vi "HFRR ADV v040 new software.vi"() -> ()   [LabVIEW 2025] (continued)
                    n2637 = Number To Fractional String(number=w3230, width (-)=i16 9 ("precision (6)"), precision (6)=i16 3) -> (F-format string=w3231:string)  [unwired: 1 in]
                    n2638 = Number To Fractional String(number=w3227, width (-)=i16 9 ("precision (6)"), precision (6)=i16 3) -> (F-format string=w3226:string)  [unwired: 1 in]
                    n2639 = Number To Fractional String(number=w3218, width (-)=i16 9 ("precision (6)"), precision (6)=i16 6) -> (F-format string=w3253:string)  [unwired: 1 in]
                    n2640 = Number To Fractional String(number=w3252, width (-)=i16 14 ("precision (6)"), precision (6)=i16 3) -> (F-format string=w3254:string)  [unwired: 1 in]
                    n2641 = Bundle("y"=1.02, "LVDT STROKE DISPLAY"=w3199, "y"=0.98) -> (w3219:T31)  [unwired: 1 in]
                    n2642 = Number To Fractional String(number="Ambient Humidity :", width (-)=i16 9 ("precision (6)"), precision (6)=i16 6) -> (F-format string=w3211:string)  [unwired: 1 in]
                    n2643 = local read "RUN"() -> (w3217:bool)
                    n2644 = case shown="True" w3217 {
                      tunnel: w3219 -> [_ w3270]
                      tunnel: w3199 -> [_ w3269]
                      tunnel: w3199 -> [_ w3267]
                      tunnel: w3199 -> [_ w3268]
                      frame False {
                      }
                      frame True {
                        "Stroke ( mm )" <- w3270
                        "Stroke ( mm )" <- w3270
                        "Stroke 4" <- w3269
                        "Stroke 3" <- w3267
                        "Stroke 2" <- w3268
                        "measured_stroke" <- w3267
                      }
                    }
                    n2645 = Concatenate Strings(w3254, w3213, w3253, w3213, w3245, w3213, w3244, w3213, w3241, w3213, w3238, w3213, w3235, w3213, w3231, w3213, w3226, w3213, w3211, "\r") -> (w3251:string)
                    n2646 = call <vilib>:"Write Characters To File.vi"("append to file? (new file:F)"=TRUE, "character string"=w3251, "file path (dialog if empty)"=w3204) -> ()  [unwired: 2 in, 1 out]
                    "refresh flag" <- TRUE ("refresh flag")
                    "LVDT STROKE Actual" <- w3197
                  }
                }
                n2647 = case shown="True" w3113 {
                  tunnel: w3123 -> [_ w3149]
                  tunnel: w3128 -> [_ w3159]
                  tunnel: [0.0 w3155] -> _
                  tunnel: w3122 -> [_ w3154]
                  tunnel: [0.0 w3153] -> _
                  tunnel: w3112 -> [_ w3153]
                  tunnel: w3126 -> [w3142 _]
                  frame False {
                    n2648 = local write "acq timer"(w3142) -> ()
                    n2649 = local write "Test Duration Status"(0.0 ("Test Duration Status")) -> ()
                  }
                  frame True {
                    n2650 = local read "Set Hz"() -> (w3156:dbl)
                    n2651 = local write "Elapsed time"(w3149) -> ()
                    n2652 = local read "test time"() -> (w3148:dbl)
                    n2653 = Multiply(x=w3159, y=w3156) -> (x*y=w3158:dbl)
                    n2654 = case shown="False" w3154 {
                      tunnel: w3158 -> [w3160 _]
                      tunnel: [w3160 1.0] -> w3155
                      frame False {
                        n2655 = local write "Cycles elapsed"(w3160) -> ()
                      }
                      frame True {
                      }
                    }
                    n2656 = Greater?(x=w3149, y=w3148) -> (0:w3157:bool)
                    n2657 = Subtract(x=w3148, y=w3149) -> (x-y=w3147:dbl)
                    n2658 = Multiply(x=w3147, y=60.0) -> (x*y=w3146:dbl)
                    n2659 = local write "Time Remaining"(w3146) -> ()
                    n2660 = local write "Remaining Time"(w3146) -> ()
                    n2661 = case shown="True" w3157 {
                      frame False {
                      }
                      frame True {
                        n2662 = stacked-sequence {
                          frame #0 {
                            w3165 = T19."Enabled" ("Disabled")
                            w3164 = FALSE ("TEST FILE NAM,E SAVED")
                            w3166 = "" ("FILE")
                            w3167 = TRUE ("Visible")
                            n2663 = local write "RUN"(FALSE ("OK Button 2")) -> ()
                            n2664 = local write "Heater Button"(FALSE ("Heater Button")) -> ()
                            n2665 = local write "Auto Start Test"(FALSE ("Auto Start Test")) -> ()
                            n2666 = local write "TestCompFlg"(TRUE ("StpFlg")) -> ()
                            n2667 = local read "Humidity ( %RH )"() -> (→"Rh After":dbl)
                            n2668 = property on="STOP 2" class="Bool (strict)"("Disabled"=u8 0) -> ()  [unwired: 2 in, 2 out]
                            n2669 = local read "EVENT LOG"() -> (w3172:string)
                            n2670 = call "Event Log.vi"("Content"="Test Completed", "EVENT LOG"=w3172) -> ("EVENT LOG"=w3171:string)  [unwired: 8 in, 1 out]
                            n2671 = property on="RUN" class="Bool (strict)"("Visible"=w3167) -> ()  [unwired: 2 in, 2 out]
                            n2672 = property on="Auto Start Test" class="Bool (strict)"("Visible"=w3167) -> ()  [unwired: 2 in, 2 out]
                            n2673 = local write "Batch Ref Num :"(w3166) -> ()
                            n2674 = local write "FILE"(w3166) -> ()
                            n2675 = local write "EVENT LOG"(w3171) -> ()
                            n2676 = local write "TEST FILE NAM,E SAVED"(w3164) -> ()
                            n2677 = local write "Fuel Discription :"(w3166) -> ()
                            n2678 = local write "START TEMP"(w3164) -> ()
                            n2679 = local write "Remarks :"(w3166) -> ()
                            n2680 = local write "Main Dashboard Buttons"(T1."Imaging" ("Main Dashboard Buttons")) -> ()
                            n2681 = local write "Main Tab"(T2."Adv Scar" ("Main Tab")) -> ()
                            n2682 = property on="FRICVALZ 2" class="Bool (strict)"("DisabledEnum"=w3165) -> ()  [unwired: 2 in, 2 out]
                            n2683 = property on="FRICVALZ 3" class="Bool (strict)"("DisabledEnum"=w3165) -> ()  [unwired: 2 in, 2 out]
                            n2684 = property on="FRICVALZ 4" class="Bool (strict)"("DisabledEnum"=w3165) -> ()  [unwired: 2 in, 2 out]
                          }
                          frame #1 {
                            n2685 = Wait (ms)(milliseconds to wait=u32 1500) -> ()  [unwired: 1 out]
                          }
                          frame #2 {
                            n2686 = local read "WriteHumidity"() -> (w3180:string[])
                            n2687 = Insert Into Array(array=w3180, new element="R;1" ("new element/subarray")) -> (w3178:string[])  [unwired: 1 in]
                            n2688 = local write "Due Write"("VC;0") -> ()
                            n2689 = local write "WriteHumidity"(w3178) -> ()
                          }
                          frame #3 {
                            n2690 = Wait (ms)(milliseconds to wait=u32 1500) -> ()  [unwired: 1 out]
                          }
                          frame #4 {
                            n2691 = local read "WriteHumidity"() -> (w3185:string[])
                            n2692 = Insert Into Array(array=w3185, new element="R;1" ("new element/subarray")) -> (w3184:string[])  [unwired: 1 in]
                            n2693 = local write "Due Write"("VC;0") -> ()
                            n2694 = local write "WriteHumidity"(w3184) -> ()
                          }
                          frame #5 {
                            n2695 = Wait (ms)(milliseconds to wait=u32 1500) -> ()  [unwired: 1 out]
                          }
                          frame #6 {
                            n2696 = local write "Due Write"("ST;0") -> ()
                          }
                          frame #7 {
                            n2697 = local write "measured_stroke"(0.0 ("measured_stroke")) -> ()
                            n2698 = Wait (ms)(milliseconds to wait=u32 1500) -> ()  [unwired: 1 out]
                          }
                          frame #8 {
                            n2699 = local write "Humidity"(FALSE ("Humidity")) -> ()
                            n2700 = local write "Due Write"("HE;0") -> ()
                          }
                          frame #9 {
                            n2701 = local write "HUMIDITY CLEAR"(TRUE ("HUMIDITY CLEAR")) -> ()
                          }
                        }
                      }
                    }
                    n2702 = Divide(x=w3149, y=w3148) -> (x/y=w3152:dbl)
                    n2703 = Multiply(x=w3152, y=100.0) -> (x*y=w3150:dbl)
                    n2704 = local write "Test Duration Status"(w3150) -> ()
                  }
                }
              }
              frame #2 {
                n2705 = case shown="True" "Heater Button" {
                  tunnel: [0.0 ("output") w3293] -> w3271
                  frame False {
                    w3274 = TRUE ("tmpchk")
                    n2706 = local read "TEMP"() -> (w3275:dbl)
                    n2707 = local write "Temp ini"(w3275) -> ()
                    n2708 = local write "Reset 4"(w3274) -> ()
                    n2709 = local write "tmpchk"(w3274) -> ()
                    n2710 = local write "reinit"(TRUE ("reinit")) -> ()
                    n2711 = local write "manual temp log"(TRUE ("manual temp log")) -> ()
                  }
                  frame True {
                    # "Logic to turn off\nthe heater when \ntemp is not rising.\nTime - 60 sec\nDelta t- 5°c"
                    n2712 = local read "Temp ini"() -> (w3282:dbl)
                    n2713 = local read "Auto Start Test"() -> (w3278:bool)
                    n2714 = Less?(x=w3282, y=53.0) -> (x < y?=w3280:bool)
                    n2715 = case shown="False" w3278 {
                      frame False {
                        n2716 = local read "Set Temp"() -> (w3302:dbl)
                        n2717 = local read "TEMP"() -> (w3301:dbl)
                        n2718 = Subtract(x=w3302, y=w3301) -> (x-y=w3300:dbl)
                        n2719 = Absolute Value(x=w3300) -> (abs(x)=w3299:dbl)
                        n2720 = Less?(x=w3299, y=0.5) -> (x < y?=w3297:bool)
                        n2721 = case shown="True" w3297 {
                          tunnel: "manual temp log" -> [_ w3303]
                          frame False {
                          }
                          frame True {
                            n2722 = case shown="True" w3303 {
                              selector: w3303 -> [_ w3304]
                              frame False {
                              }
                              frame True {
                                # "#Event log"
                                n2723 = Not(x=w3304) -> (.not. x?=w3305:bool)
                                n2724 = local write "manual temp log"(w3305) -> ()
                                n2725 = local read "EVENT LOG"() -> (w3308:string)
                                n2726 = call "Event Log.vi"("Content"="Target Temperature reached", "EVENT LOG"=w3308) -> ("EVENT LOG"=w3307:string)  [unwired: 8 in, 1 out]
                                n2727 = local write "EVENT LOG"(w3307) -> ()
                              }
                            }
                          }
                        }
                      }
                      frame True {
                        n2728 = local write "manual temp log"(TRUE ("manual temp log")) -> ()
                      }
                    }
                    n2729 = And(x="tmpchk", y=w3280) -> (x .and. y?=w3283:bool)
                    n2730 = case shown="True" w3283 {
                      frame False {
                      }
                      frame True {
                        n2731 = call "Elapsed Time8"("Time Target (s)"=300.0, "Reset"="Reset 4") -> ("Time has Elapsed"=w3310:bool)  [unwired: 10 in, 7 out]
                        n2732 = flat-sequence {
                          tunnel: w3310 -> [_]
                          frame #0 {
                            n2733 = local write "Reset 4"(FALSE ("Reset 4")) -> ()
                          }
                        }
                        n2734 = case shown="True" w3310 {
                          frame False {
                          }
                          frame True {
                            n2735 = local read "Temp ini"() -> (w3317:dbl)
                            n2736 = Add(x=w3317, y=5.0) -> (x+y=w3315:dbl)
                            n2737 = local read "TEMP"() -> (w3318:dbl)
                            n2738 = Greater?(x=w3318, y=w3315) -> (0:w3316:bool)
                            n2739 = case shown="False" w3316 {
                              frame False {
                                n2740 = local write "Heater Button"(FALSE ("Heater Button")) -> ()
                              }
                              frame True {
                                n2741 = local write "tmpchk"(FALSE ("tmpchk")) -> ()
                              }
                            }
                          }
                        }
                      }
                    }
                    n2742 = local read "Set Temp"() -> (w3291:dbl)
                    n2743 = local read "TEMP"() -> (w3285:dbl)
                    n2744 = call-poly <vilib>:"PID.vi"("reinitialize? (F)"="reinit", "dt (s)"=-1.0, "process variable"=w3285, "setpoint"=w3291) -> ("output"=w3288:dbl)  [unwired: 6 in, 1 out]
                    n2745 = Subtract(x=w3291, y=w3285) -> (x-y=w3292:dbl)
                    n2746 = Add(x=w3291, y=0.5) -> (x+y=w3289:dbl)
                    n2747 = Greater Or Equal?(x=w3285, y=w3289) -> ()  [unwired: 1 out]
                    n2748 = Select(t=0.0, s=FALSE, f=w3288) -> (s? t:f=w3287:dbl)
                    "PID output" <- w3287
                    n2749 = flat-sequence {
                      tunnel: w3287 -> [w3321]
                      tunnel: [w3321] -> w3293
                      frame #0 {
                        n2750 = local write "reinit"(FALSE ("reinit")) -> ()
                      }
                    }
                    n2751 = Bundle(w3292, "output"=w3287, "TEMP"=w3285) -> ()  [unwired: 1 in, 1 out]
                  }
                }
                "PID-out" <- w3271
              }
              frame #3 {
                n2752 = local read "TEMP"() -> (w3323:dbl)
                n2753 = Greater Or Equal?(x=w3323, y="Set Temp 2") -> (x >= y?=w3328:bool)
                n2754 = case shown="True" w3328 {
                  tunnel: [FALSE TRUE] -> w3326
                  frame False {
                  }
                  frame True {
                  }
                }
                "Status 13" <- w3326
                n2755 = And(x=w3326, y="trip1 8") -> (x .and. y?=w3325:bool)
                n2756 = case shown="True" w3325 {
                  frame False {
                    n2757 = local write "Heater Trip Temp"(TRUE ("Heater Trip Temp")) -> ()
                  }
                  frame True {
                    w3331 = FALSE ("OK Button 2")
                    n2758 = case shown="True" "Heater Trip Temp" {
                      selector: "Heater Trip Temp" -> [_ w3333]
                      frame False {
                      }
                      frame True {
                        n2759 = Not(x=w3333) -> (.not. x?=w3332:bool)
                        n2760 = local read "EVENT LOG"() -> (w3336:string)
                        n2761 = local write "Heater Trip Temp"(w3332) -> ()
                        n2762 = call "Event Log.vi"("Content"="Heater Trip", "EVENT LOG"=w3336) -> ("EVENT LOG"=w3335:string)  [unwired: 8 in, 1 out]
                        n2763 = local write "EVENT LOG"(w3335) -> ()
                      }
                    }
                    n2764 = local write "RUN"(w3331) -> ()
                    n2765 = property on="Auto Start Test" class="Bool (strict)"("Value"=w3331) -> ()  [unwired: 2 in, 2 out]
                    n2766 = local write "Heater Button"(w3331) -> ()
                  }
                }
              }
            }
            n2767 = case shown="False" w3037 {
              frame False {
                n2768 = disable-structure shown="Disabled" {
                  frame Disabled {
                    n2769 = stacked-sequence {
                      frame #0 {
                        n2770 = local write "RUN"(FALSE ("OK Button 2")) -> ()
                      }
                      frame #1 {
                      }
                    }
                  }
                  frame Enabled {
                  }
                }
              }
              frame True {
              }
            }
          }
        }
        n2771 = local read "Reset Graph"() -> (w2930:bool)
        n2772 = case shown="True" w2930 {
          selector: w2930 -> [_ w2947]
          frame False {
          }
          frame True {
            w2961 = 0.0 ("X Scale.Range:Maximum")
            n2773 = Not(x=w2947) -> (.not. x?=w2946:bool)
            n2774 = local write "Reset Graph"(w2946) -> ()
            n2775 = property on="Electrical Contact Resistance ( % )" class="WFChart (strict)"("XScale.Maximum"=600.0 ("X Scale.Range:Maximum"), "XScale.Minimum"=0.0 ("X Scale.Range:Minimum"), "YScale.Maximum"=100.0 ("Y Scale.Range:Maximum"), "YScale.Minimum"=0.0 ("Y Scale.Range:Minimum")) -> ()  [unwired: 2 in, 2 out]
            n2776 = property on="Frictional Force ( N )" class="WFChart (strict)"("XScale.Maximum"=600.0 ("X Scale.Range:Maximum"), "XScale.Minimum"=0.0 ("X Scale.Range:Minimum"), "YScale.Maximum"=100.0 ("Y Scale.Range:Maximum"), "YScale.Minimum"=0.0 ("Y Scale.Range:Minimum")) -> ()  [unwired: 2 in, 2 out]
            n2777 = property on="Temperature ( Deg C )" class="WFChart (strict)"("XScale.Maximum"=600.0 ("X Scale.Range:Maximum"), "XScale.Minimum"=0.0 ("X Scale.Range:Minimum"), "YScale.Maximum"=100.0 ("Y Scale.Range:Maximum"), "YScale.Minimum"=0.0 ("Y Scale.Range:Minimum")) -> ()  [unwired: 2 in, 2 out]
            n2778 = property on="Stroke ( mm )" class="WFChart (strict)"("XScale.Maximum"=600.0 ("X Scale.Range:Maximum"), "XScale.Minimum"=0.0 ("X Scale.Range:Minimum"), "YScale.Maximum"=100.0 ("Y Scale.Range:Maximum"), "YScale.Minimum"=0.0 ("Y Scale.Range:Minimum")) -> ()  [unwired: 2 in, 2 out]
            n2779 = property on="Coefficient of Friction" class="WFChart (strict)"("XScale.Maximum"=600.0 ("X Scale.Range:Maximum"), "XScale.Minimum"=0.0 ("X Scale.Range:Minimum"), "YScale.Maximum"=100.0 ("Y Scale.Range:Maximum"), "YScale.Minimum"=0.0 ("Y Scale.Range:Minimum")) -> ()  [unwired: 2 in, 2 out]
            n2780 = property on="Electrical Contact Resistance ( % )" class="WFChart (strict)"("XScale.Minimum"=0.0 ("X Scale.Range:Minimum"), "XScale.Maximum"=600.0 ("X Scale.Range:Maximum"), "YScale.Minimum"=0.0 ("Y Scale.Range:Minimum"), "YScale.Maximum"=100.0 ("Y Scale.Range:Maximum")) -> ()  [unwired: 2 in, 2 out]
            n2781 = property on="Temperature ( Deg C )" class="WFChart (strict)"("XScale.Minimum"=0.0 ("X Scale.Range:Minimum"), "XScale.Maximum"=600.0 ("X Scale.Range:Maximum"), "YScale.Minimum"=0.0 ("Y Scale.Range:Minimum"), "YScale.Maximum"=100.0 ("Y Scale.Range:Maximum")) -> ()  [unwired: 2 in, 2 out]
            n2782 = property on="Coefficient of Friction" class="WFChart (strict)"("XScale.Minimum"=0.0 ("X Scale.Range:Minimum"), "XScale.Maximum"=600.0 ("X Scale.Range:Maximum"), "YScale.Maximum"=1.0 ("X Scale.Range:Minimum"), "YScale.Minimum"=0.0 ("X Scale.Range:Minimum")) -> ()  [unwired: 2 in, 2 out]
            n2783 = property on="Frictional Force ( N )" class="WFChart (strict)"("XScale.Maximum"=600.0 ("X Scale.Range:Maximum"), "XScale.Minimum"=w2961, "YScale.Maximum"=10.0 ("Y Scale.Range:Maximum"), "YScale.Minimum"=w2961) -> ()  [unwired: 2 in, 2 out]
            n2784 = property on="Stroke ( mm )" class="WFChart (strict)"("XScale.Maximum"=600.0 ("X Scale.Range:Maximum"), "XScale.Minimum"=0.0 ("X Scale.Range:Minimum"), "YScale.Maximum"=100.0 ("Y Scale.Range:Maximum"), "YScale.Minimum"=0.0 ("Y Scale.Range:Minimum")) -> ()  [unwired: 2 in, 2 out]
            n2785 = property on="Humidity ( %RH ) 2" class="WFChart (strict)"("XScale.Maximum"=600.0 ("X Scale.Range:Maximum"), "XScale.Minimum"=0.0 ("X Scale.Range:Minimum"), "YScale.Maximum"=100.0 ("Y Scale.Range:Maximum"), "YScale.Minimum"=0.0 ("Y Scale.Range:Minimum")) -> ()  [unwired: 2 in, 2 out]
          }
        }
      }
      frame "Compare Files" {
        # "Elapsed time\ncof\nstroke\nAir temp\nTemp\nHumidity"
        n2786 = case shown="True" "RSTV1 2" {
          frame False {
          }
          frame True {
            n2787 = property on="Humidity ( %RH )" class="XYGraph (strict)"("Y Scale.Display Format:Precision"=u8 0 ("Y Scale.Format & Precision:Precision")) -> ()  [unwired: 2 in, 2 out]
            n2788 = property on="Humidity ( %RH )" class="XYGraph (strict)"("X Scale.Range:Minimum"=0.0, "X Scale.Range:Maximum"=75.0, "Y Scale.Range:Minimum"=48.0, "Y Scale.Range:Maximum"=58.0) -> ()  [unwired: 2 in, 2 out]
          }
        }
        n2789 = case shown="True" "RST CP 2" {
          frame False {
          }
          frame True {
            n2790 = property on="XY Graph 13" class="XYGraph (strict)"("Y Scale.Display Format:Precision"=u8 0 ("Y Scale.Format & Precision:Precision")) -> ()  [unwired: 2 in, 2 out]
            n2791 = property on="XY Graph 13" class="XYGraph (strict)"("X Scale.Range:Minimum"=0.0, "X Scale.Range:Maximum"=75.0, "Y Scale.Range:Minimum"=0.0, "Y Scale.Range:Maximum"=100.0) -> ()  [unwired: 2 in, 2 out]
          }
        }
        n2792 = case shown="True" "RST CP" {
          frame False {
          }
          frame True {
            n2793 = property on="Sample Temperature ( °C )" class="XYGraph (strict)"("Y Scale.Display Format:Precision"=u8 2 ("Y Scale.Format & Precision:Precision")) -> ()  [unwired: 2 in, 2 out]
            n2794 = property on="Sample Temperature ( °C )" class="XYGraph (strict)"("X Scale.Range:Minimum"=0.0, "X Scale.Range:Maximum"=75.0, "Y Scale.Range:Minimum"=58.0, "Y Scale.Range:Maximum"=62.0) -> ()  [unwired: 2 in, 2 out]
          }
        }
        n2795 = case shown="True" "RSTV1 3" {
          frame False {
          }
          frame True {
            n2796 = property on="Air Temperature  ( °C )" class="XYGraph (strict)"("Y Scale.Display Format:Precision"=u8 2 ("Y Scale.Format & Precision:Precision")) -> ()  [unwired: 2 in, 2 out]
            n2797 = property on="Air Temperature  ( °C )" class="XYGraph (strict)"("X Scale.Range:Minimum"=0.0 ("Y Scale.Range:Minimum"), "X Scale.Range:Maximum"=75.0 ("Y Scale.Range:Maximum"), "Y Scale.Range:Minimum"=20.0 ("X Scale.Range:Minimum"), "Y Scale.Range:Maximum"=26.0 ("X Scale.Range:Maximum")) -> ()  [unwired: 2 in, 2 out]
          }
        }
        n2798 = case shown="True" "RSTV1 4" {
          frame False {
          }
          frame True {
            n2799 = property on="Stroke ( mm )" class="XYGraph (strict)"("Y Scale.Display Format:Precision"=u8 2 ("Y Scale.Format & Precision:Precision")) -> ()  [unwired: 2 in, 2 out]
            n2800 = property on="Stroke ( mm )" class="XYGraph (strict)"("X Scale.Range:Minimum"=0.0 ("Y Scale.Range:Maximum"), "X Scale.Range:Maximum"=75.0 ("X Scale.Range:Minimum"), "Y Scale.Range:Minimum"=0.98, "Y Scale.Range:Maximum"=1.02) -> ()  [unwired: 2 in, 2 out]
          }
        }
        n2801 = case shown="True" "rstv2" {
          frame False {
          }
          frame True {
            n2802 = property on="Coefficient Of Friction" class="XYGraph (strict)"("Y Scale.Display Format:Precision"=u8 3 ("Y Scale.Format & Precision:Precision")) -> ()  [unwired: 2 in, 2 out]
            n2803 = property on="Coefficient Of Friction" class="XYGraph (strict)"("X Scale.Range:Minimum"=0.0 ("Y Scale.Range:Maximum"), "X Scale.Range:Maximum"=75.0, "Y Scale.Range:Minimum"=0.0, "Y Scale.Range:Maximum"=1.0 ("X Scale.Range:Minimum")) -> ()  [unwired: 2 in, 2 out]
          }
        }
        n2804 = case shown="True" "RST CP 3" {
          frame False {
          }
          frame True {
            n2805 = property on="Air Temp ( °C ) vs Humidity ( % RH )" class="XYGraph (strict)"("X Scale.Range:Minimum"=18.0, "X Scale.Range:Maximum"=28.0 ("X Scale.Range:Minimum"), "Y Scale.Range:Minimum"=30.0 ("X Scale.Range:Minimum"), "Y Scale.Range:Maximum"=70.0 ("X Scale.Range:Minimum")) -> ()  [unwired: 2 in, 2 out]
          }
        }
        n2806 = case shown="True" "OPEN 1" {
          frame False {
          }
          frame True {
            (unwired) 0  # existing file
            w3612 = "Choose a datalog file to open"  # prompt
            n2807 = local write "OPEN 1"(FALSE ("OPEN 1")) -> ()
            n2808 = String To Path(string="C:\\LAB-IQ\\Data\\") -> (path=w3597:path)
            n2809 = File Dialog(6:"*.dgf" ("pattern"), 7:w3612, 11:w3597) -> (0:w3595:errorcluster, 3:w3603:path)  [unwired: 4 in, 2 out]
            n2810 = Unbundle(w3595) -> ()  [unwired: 3 out]
            n2811 = Strip Path(path=w3603) -> (name=w3602:string)  [unwired: 1 out]
            n2812 = Path To String(path=w3603) -> (string=w3598:string)
            "string1" <- w3598
            n2813 = Match Pattern(string=w3602, regular expression=".dgf") -> (before substring=→"String Control":string)  [unwired: 1 in, 3 out]
            n2814 = Match Pattern(string=w3598, regular expression=".dgf" ("substring (\"\")")) -> (before substring=w3608:string)  [unwired: 1 in, 3 out]
            n2815 = Concatenate Strings(w3608, ".duf" ("Substring")) -> (w3604:string)
            n2816 = String To Path(string=w3604) -> (path=w3609:path)
            n2817 = call <vilib>:"Read Characters From File.vi"("file path (dialog if empty)"=w3609, "start of read offset (chars.:0)"=60 ("start of read offset (chars.: 0)")) -> ("character string"=→"String Control 2":string)  [unwired: 4 in, 3 out]
          }
        }
        n2818 = case shown="True" "OPEN 2" {
          frame False {
          }
          frame True {
            (unwired) 0  # existing file
            w3630 = "Choose a datalog file to open"  # prompt
            n2819 = local write "OPEN 2"(FALSE ("OPEN 1")) -> ()
            n2820 = String To Path(string="C:\\LAB-IQ\\Data\\") -> (path=w3615:path)
            n2821 = File Dialog(6:"*.dgf" ("pattern"), 7:w3630, 11:w3615) -> (0:w3613:errorcluster, 3:w3621:path)  [unwired: 4 in, 2 out]
            n2822 = Unbundle(w3613) -> ()  [unwired: 3 out]
            n2823 = Strip Path(path=w3621) -> (name=w3619:string)  [unwired: 1 out]
            n2824 = Path To String(path=w3621) -> (string=w3616:string)
            "string1 2" <- w3616
            n2825 = Match Pattern(string=w3619, regular expression=".dgf") -> (before substring=→"String Control 3":string)  [unwired: 1 in, 3 out]
            n2826 = Match Pattern(string=w3616, regular expression=".dgf" ("substring (\"\")")) -> (before substring=w3627:string)  [unwired: 1 in, 3 out]
            n2827 = Concatenate Strings(w3627, ".duf" ("Substring")) -> (w3624:string)
            n2828 = String To Path(string=w3624) -> (path=w3622:path)
            n2829 = call <vilib>:"Read Characters From File.vi"("file path (dialog if empty)"=w3622, "start of read offset (chars.:0)"=60 ("start of read offset (chars.: 0)")) -> ("character string"=→"String Control 4":string)  [unwired: 4 in, 3 out]
          }
        }
        n2830 = case shown="True" "OPEN 3" {
          frame False {
          }
          frame True {
            (unwired) 0  # existing file
            w3648 = "Choose a datalog file to open"  # prompt
            n2831 = local write "OPEN 3"(FALSE ("OPEN 1")) -> ()
            n2832 = String To Path(string="C:\\LAB-IQ\\Data\\") -> (path=w3633:path)
            n2833 = File Dialog(6:"*.dgf" ("pattern"), 7:w3648, 11:w3633) -> (0:w3631:errorcluster, 3:w3639:path)  [unwired: 4 in, 2 out]
            n2834 = Unbundle(w3631) -> ()  [unwired: 3 out]
            n2835 = Strip Path(path=w3639) -> (name=w3637:string)  [unwired: 1 out]
            n2836 = Path To String(path=w3639) -> (string=w3634:string)
            "string1 3" <- w3634
            n2837 = Match Pattern(string=w3637, regular expression=".dgf") -> (before substring=→"String Control 5":string)  [unwired: 1 in, 3 out]
            n2838 = Match Pattern(string=w3634, regular expression=".dgf" ("substring (\"\")")) -> (before substring=w3644:string)  [unwired: 1 in, 3 out]
            n2839 = Concatenate Strings(w3644, ".duf" ("Substring")) -> (w3641:string)
            n2840 = String To Path(string=w3641) -> (path=w3645:path)
            n2841 = call <vilib>:"Read Characters From File.vi"("file path (dialog if empty)"=w3645, "start of read offset (chars.:0)"=60 ("start of read offset (chars.: 0)")) -> ("character string"=→"String Control 6":string)  [unwired: 4 in, 3 out]
          }
        }
        n2842 = case shown="True" "OPEN 4" {
          frame False {
          }
          frame True {
            (unwired) 0  # existing file
            w3666 = "Choose a datalog file to open"  # prompt
            n2843 = local write "OPEN 4"(FALSE ("OPEN 1")) -> ()
            n2844 = String To Path(string="C:\\LAB-IQ\\Data\\") -> (path=w3651:path)
            n2845 = File Dialog(6:"*.dgf" ("pattern"), 7:w3666, 11:w3651) -> (0:w3649:errorcluster, 3:w3657:path)  [unwired: 4 in, 2 out]
            n2846 = Unbundle(w3649) -> ()  [unwired: 3 out]
            n2847 = Strip Path(path=w3657) -> (name=w3655:string)  [unwired: 1 out]
            n2848 = Path To String(path=w3657) -> (string=w3652:string)
            "string1 4" <- w3652
            n2849 = Match Pattern(string=w3655, regular expression=".dgf") -> (before substring=→"String Control 7":string)  [unwired: 1 in, 3 out]
            n2850 = Match Pattern(string=w3652, regular expression=".dgf" ("substring (\"\")")) -> (before substring=w3662:string)  [unwired: 1 in, 3 out]
            n2851 = Concatenate Strings(w3662, ".duf" ("Substring")) -> (w3659:string)
            n2852 = String To Path(string=w3659) -> (path=w3663:path)
            n2853 = call <vilib>:"Read Characters From File.vi"("file path (dialog if empty)"=w3663, "start of read offset (chars.:0)"=60 ("start of read offset (chars.: 0)")) -> ("character string"=→"String Control 8":string)  [unwired: 4 in, 3 out]
          }
        }
      }
      frame "About" {
        # "Elapsed time\ncof\nstroke\nmean pos\nTemp\nHumidity"
        n2854 = disable-structure shown="Disabled" {
          frame Disabled {
            n2855 = case shown="True" "Export" {
              frame False {
              }
              frame True {
                w3688 = "                                      " ("string")
                w3690 = "\r"
                (unwired) i16 6 ("width (-)")
                w3767 = "\r"
                w3699 = "\r"
                n2856 = local write "Export"(FALSE ("Export")) -> ()
                n2857 = local read "String 29"() -> (w3736:string)
                n2858 = local read "String 34"() -> (w3724:string)
                n2859 = local read "String 35"() -> (w3719:string)
                n2860 = local read "String 37"() -> (w3715:string)
                n2861 = local read "String 36"() -> (w3712:string)
                n2862 = local read "String 38"() -> (w3709:string)
                n2863 = local read "String 39"() -> (w3706:string)
                n2864 = Match Pattern(string=w3736, regular expression=".dwm") -> (before substring=w3732:string)  [unwired: 1 in, 3 out]
                "before substring" <- w3732
                n2865 = local read "S 38"() -> (w3727:string)
                n2866 = local read "S 39"() -> (w3720:string)
                n2867 = local read "Temperature before test 2"() -> (w3756:dbl)
                n2868 = local read "Temperature after test 2"() -> (w3761:dbl)
                n2869 = local read "Humidity before test 2"() -> (w3742:dbl)
                n2870 = local read "Humidity after test 2"() -> (w3757:dbl)
                n2871 = local read "MWSD 2"() -> (w3753:dbl)
                n2872 = local read "WS1.4 2"() -> (w3769:dbl)
                n2873 = local read "HCF 2"() -> (w3765:dbl)
                n2874 = local read "AVP 2"() -> (w3754:dbl)
                n2875 = Concatenate Strings("1," ("string"), w3727) -> (w3726:string)
                n2876 = Concatenate Strings("2," ("string"), w3724) -> (w3723:string)
                n2877 = Concatenate Strings("3," ("string"), w3720) -> (w3722:string)
                n2878 = Concatenate Strings("4," ("string"), w3719) -> (w3718:string)
                n2879 = Concatenate Strings("5," ("string"), w3715) -> (w3716:string)
                n2880 = Concatenate Strings("6," ("string"), w3712) -> (w3713:string)
                n2881 = Concatenate Strings("7," ("string"), w3709) -> (w3710:string)
                n2882 = Concatenate Strings("8," ("string"), w3706) -> (w3707:string)
                n2883 = local read "Sample ID"() -> (w3774:string)
                n2884 = case shown="\"xlx\"" "Select File Type" {
                  tunnel: w3732 -> [w3777 w3779 w3781]
                  tunnel: [w3775 w3780 w3782] -> w3731
                  frame "xlx" {
                    n2885 = Concatenate Strings(w3777, ".xls" ("string")) -> (w3775:string)
                  }
                  frame "csv" {
                    n2886 = Concatenate Strings(w3779, ".csv" ("string")) -> (w3780:string)
                  }
                  frame "txt" {
                    n2887 = Concatenate Strings(w3781, ".txt" ("string")) -> (w3782:string)
                  }
                }
                n2888 = local read "Test Date"() -> (w3773:string)
                n2889 = local read "String 45"() -> (w3687:string)
                n2890 = local read "String 31"() -> (w3772:string)
                n2891 = local read "String 32"() -> (w3771:string)
                n2892 = local read "TITTLE"() -> (w3695:string)
                n2893 = Number To Fractional String(number=w3742, width (-)=i16 6, precision (6)=i16 2) -> (F-format string=w3741:string)  [unwired: 1 in]
                n2894 = Number To Fractional String(number=w3756, width (-)=i16 6, precision (6)=i16 2) -> (F-format string=w3762:string)  [unwired: 1 in]
                n2895 = Number To Fractional String(number=w3757, width (-)=i16 6, precision (6)=i16 2) -> (F-format string=w3755:string)  [unwired: 1 in]
                n2896 = Number To Fractional String(number=w3761, width (-)=i16 6, precision (6)=i16 2) -> (F-format string=w3760:string)  [unwired: 1 in]
                n2897 = Number To Fractional String(number=w3753, width (-)=i16 6, precision (6)=i16 2) -> (F-format string=w3751:string)  [unwired: 1 in]
                n2898 = Number To Fractional String(number=w3754, width (-)=i16 6, precision (6)=i16 2) -> (F-format string=w3752:string)  [unwired: 1 in]
                n2899 = Number To Fractional String(number=w3765, width (-)=i16 6, precision (6)=i16 2) -> (F-format string=w3766:string)  [unwired: 1 in]
                n2900 = Number To Fractional String(number=w3769, precision (6)=i16 2) -> (F-format string=w3770:string)  [unwired: 2 in]
                n2901 = local read "s.NO"() -> (w3689:string)
                n2902 = Concatenate Strings("=" ("string"), w3695) -> (w3694:string)
                n2903 = Concatenate Strings("S.No," ("string"), "                                       Parameters" ("string")) -> (w3700:string)
                n2904 = Concatenate Strings(w3767, w3726, w3741, w3767, w3723, w3762, w3767, w3722, w3755, w3767, w3718, w3760, w3767, w3716, w3751, w3767, w3713, w3752, w3767, w3710, w3766, w3767, w3707, w3770) -> (w3729:string)
                n2905 = Concatenate Strings(w3699, "," ("string"), w3687, w3689, w3688, w3771, w3774, w3688, w3772, w3773, w3699) -> (w3697:string)
                n2906 = local read "Tested by"() -> (w3703:string)
                n2907 = local read "String 33"() -> (w3704:string)
                n2908 = Concatenate Strings("," ("string"), "                                                                             " ("string")) -> (w3692:string)
                n2909 = Concatenate Strings(w3694, w3690, w3697, w3690, w3700, w3729, w3690, w3692, w3704, w3703) -> (→"export":string)
                n2910 = String To Path(string=w3731) -> (path=w3738:path)
                n2911 = local read "export"() -> (w3733:string)
                n2912 = call <vilib>:"Write Characters To File.vi"("append to file? (new file:F)"=FALSE, "character string"=w3733, "file path (dialog if empty)"=w3738) -> ()  [unwired: 2 in, 1 out]
              }
            }
          }
          frame Enabled {
          }
        }
        n2913 = case shown="True" "OK Button 17" {
          frame False {
          }
          frame True {
            (unwired) 0  # existing file
            w3991 = "Choose a datalog file to open"  # prompt
            n2914 = local write "OK Button 17"(FALSE ("OK Button 17")) -> ()
            n2915 = local read "String"() -> (w3986:string)
            n2916 = String To Path(string=w3986) -> (path=w3987:path)
            n2917 = File Dialog(6:"*.duf" ("pattern"), 7:w3991, 11:w3987) -> (0:w3978:errorcluster, 3:w3997:path)  [unwired: 4 in, 2 out]
            n2918 = Unbundle(w3978) -> ()  [unwired: 3 out]
            n2919 = Open/Create/Replace File "Open File"(file path (use dialog)=w3997) -> (refnum out=w3989:refnum<file>)  [unwired: 5 in, 2 out]
            n2920 = Strip Path(path=w3997) -> (name=w3995:string)  [unwired: 1 out]
            n2921 = Path To String(path=w3997) -> (string=w3980:string)
            n2922 = while {
              tunnel: w3989 -> [w4001]
              i -> [w3998]
              stop <- w3999 continue-if-true
              (unwired) TRUE ("line mode (F)")
              n2923 = Read from Text File "Read File"(file (use dialog)=w4001) -> (text=w4000:string)  [unwired: 3 in, 3 out]
              n2924 = local write "Numeric 16"(w3998) -> ()
              n2925 = String Length(string=w4000) -> (length=w4003:i32)
              n2926 = Greater?(x=w4003, y=1) -> (0:w3999:bool)
            }
            n2927 = local write "String 29"(w3980) -> ()
            n2928 = Search and Replace String(input string=w3980, search string=".duf", replace string=".dgf" ("replace string (\"\")")) -> (result string=→"String Indicator 4":string)  [unwired: 5 in, 3 out]
            n2929 = Match Pattern(string=w3995, regular expression=".dwm") -> (before substring=w3979:string)  [unwired: 1 in, 3 out]
            "String Indicator" <- w3979
            n2930 = Match Pattern(string=w3980, regular expression=".dwm" ("substring (\"\")")) -> (before substring=w3981:string)  [unwired: 1 in, 3 out]
            "String Indicator 3" <- w3981
            n2931 = local write "TITTLE 2"(w3979) -> ()
            n2932 = String To Path(string=w3981) -> (path=w3988:path)
            "path" <- w3988
            n2933 = call <vilib>:"Read Characters From File.vi"("file path (dialog if empty)"=w3988, "start of read offset (chars.:0)"=60 ("start of read offset (chars.: 0)")) -> ("character string"=→"String Indicator 2":string)  [unwired: 4 in, 3 out]
          }
        }
        n2934 = call <vilib>:"Query Available Printers.vi"() -> ("system configured printers"=w3680:string[])  [unwired: 9 in, 2 out]
        "System Configured Printers 2" <- w3680
        n2935 = local read "OK Button 16"() -> (w3677:bool)
        n2936 = case shown="True" "OK Button 16" {
          frame False {
          }
          frame True {
            n2937 = stacked-sequence {
              frame #0 {
                n2938 = local read "Numeric 16"() -> (w4005:i32)
                n2939 = local write "Numeric 10"(w4005) -> ()
              }
              frame #1 {
                n2940 = local read "String 29"() -> (w4008:string)
                n2941 = String To Path(string=w4008) -> (path=w4007:path)
                n2942 = Open/Create/Replace File "Open File"(file path (use dialog)=w4007) -> (refnum out=w4009:refnum<file>)  [unwired: 5 in, 2 out]
                n2943 = for {
                  N: 16 -> [_]
                  tunnel: w4009 -> [w4016]
                  i -> [w4012]
                  (unwired) TRUE ("line mode (F)")
                  n2944 = Read from Text File "Read File"(file (use dialog)=w4016) -> (text=w4010:string)  [unwired: 3 in, 3 out]
                  n2945 = Match Pattern(string=w4010, regular expression="(") -> (after substring=w4015:string)  [unwired: 1 in, 3 out]
                  n2946 = Match Pattern(string=w4015, regular expression=")") -> (before substring=w4011:string)  [unwired: 1 in, 3 out]
                  n2947 = case shown="1" w4012 {
                    tunnel: w4011 -> [w4017 w4018 _ _ w4019 w4020 w4021 w4023 w4025 w4027 w4029 w4031 w4033 w4035 _]
                    tunnel: w4010 -> [_ _ _ _ _ _ _ _ _ _ _ _ _ _ _]
                    frame 0 {
                      "TITTLE" <- w4017
                    }
                    frame 1 {
                      "Sample ID" <- w4018
                    }
                    frame 2 {
                    }
                    frame 3 {
                    }
                    frame 4 {
                      "Test Date" <- w4019
                    }
                    frame 5 {
                      "Tested by" <- w4020
                    }
                    frame 6 {
                      n2948 = Fract/Exp String To Number(string=w4021) -> (number=→"Humidity before test 2":dbl)  [unwired: 3 in, 1 out]
                    }
                    frame 7 {
                      n2949 = Fract/Exp String To Number(string=w4023) -> (number=→"Temperature before test 2":dbl)  [unwired: 3 in, 1 out]
                    }
                    frame 8 {
                      n2950 = Fract/Exp String To Number(string=w4025) -> (number=→"Humidity after test 2":dbl)  [unwired: 3 in, 1 out]
                    }
                    frame 9 {
                      n2951 = Fract/Exp String To Number(string=w4027) -> (number=→"Temperature after test 2":dbl)  [unwired: 3 in, 1 out]
                    }
                    frame 10 {
                      n2952 = Fract/Exp String To Number(string=w4029) -> (number=→"MWSD 2":dbl)  [unwired: 3 in, 1 out]
                    }
                    frame 11 {
                      n2953 = Fract/Exp String To Number(string=w4031) -> (number=→"AVP 2":dbl)  [unwired: 3 in, 1 out]
                    }
                    frame 12 {
                      n2954 = Fract/Exp String To Number(string=w4033) -> (number=→"HCF 2":dbl)  [unwired: 3 in, 1 out]
                    }
                    frame 13 {
                      n2955 = Fract/Exp String To Number(string=w4035) -> (number=→"WS1.4 2":dbl)  [unwired: 3 in, 1 out]
                    }
                    frame 14, Default {
                    }
                  }
                }
              }
              frame #2 {
              }
            }
            n2956 = local write "OK Button 16"(FALSE ("OK Button 13")) -> ()
          }
        }
        n2957 = Index Array(array=w3680, index="Select Printer 3") -> (element=w3682:string)
        "Selected Printer" <- w3682
        n2958 = case shown="True" w3677 {
          frame False {
          }
          frame True {
            n2959 = flat-sequence {
              frame #0 {
              }
              frame #1 {
                n2960 = Wait (ms)(milliseconds to wait=u32 100) -> ()  [unwired: 1 out]
              }
              frame #2 {
                n2961 = local write "OK Button 16"(FALSE ("Print 3")) -> ()
              }
            }
          }
        }
        n2962 = case shown="True" "Print" {
          tunnel: w3682 -> [_ w3974]
          frame False {
          }
          frame True {
            (unwired) i16 6 ("width (-)")
            (unwired) "TESTED BY : "
            (unwired) "TESTED DATE :"
            (unwired) "SAMPLE ID : "
            (unwired) "SAMPLE DESIGN : "
            w3932 = "\r"
            w3949 = "\r"
            # "add image"
            n2963 = local read "Sample ID"() -> (w3922:string)
            n2964 = local read "Tested by"() -> (w3925:string)
            n2965 = local read "String 34"() -> (w3912:string)
            n2966 = local read "String 45"() -> (w3892:string)
            n2967 = local read "String 35"() -> (w3907:string)
            n2968 = local read "String 37"() -> (w3905:string)
            n2969 = local read "String 32"() -> (w3927:string)
            n2970 = local read "String 36"() -> (w3902:string)
            n2971 = local read "String 31"() -> (w3926:string)
            n2972 = local read "Test Date"() -> (w3923:string)
            n2973 = local read "String 33"() -> (w3928:string)
            n2974 = local read "String 38"() -> (w3898:string)
            n2975 = local read "String 39"() -> (w3895:string)
            n2976 = local write "Print"(FALSE ("Print FF")) -> ()
            n2977 = local read "S 39"() -> (w3910:string)
            n2978 = local read "S 38"() -> (w3917:string)
            n2979 = local read "Temperature before test 2"() -> (w3948:dbl)
            n2980 = local read "Temperature after test 2"() -> (w3938:dbl)
            n2981 = local read "Humidity before test 2"() -> (w3963:dbl)
            n2982 = local read "Humidity after test 2"() -> (w3947:dbl)
            n2983 = local read "MWSD 2"() -> (w3952:dbl)
            n2984 = local read "WS1.4 2"() -> (w3930:dbl)
            n2985 = Concatenate Strings("2)" ("string"), w3912) -> (w3913:string)
            n2986 = Concatenate Strings("3)" ("string"), w3910) -> (w3911:string)
            n2987 = Concatenate Strings("1)" ("string"), w3917) -> (w3916:string)
            n2988 = Concatenate Strings("4)" ("string"), w3907) -> (w3908:string)
            n2989 = Concatenate Strings("5)" ("string"), w3905) -> (w3904:string)
            n2990 = Concatenate Strings("6)" ("string"), w3902) -> (w3901:string)
            n2991 = Concatenate Strings("7)" ("string"), w3898) -> (w3899:string)
            n2992 = Concatenate Strings("8)" ("string"), w3895) -> (w3896:string)
            n2993 = local read "HCF 2"() -> (w3934:dbl)
            n2994 = local read "AVP 2"() -> (w3951:dbl)
            n2995 = local read "s.NO"() -> (w3893:string)
            n2996 = call <vilib>:"New Report.vi"("report type"=enum16{"Standard Report", "HTML"}."Standard Report") -> ("report out"=w3972:refnum<class "NI_report.lvclass">, "error out"=w3971:errorcluster)  [unwired: 13 in]
            n2997 = local read "TITTLE"() -> (w3924:string)
            n2998 = Concatenate Strings(w3949, w3892, w3893, w3949, w3927, w3922, w3949, w3926, w3923, w3949, w3928, w3925, w3949) -> (w3942:string)
            "test by" <- w3942
            n2999 = Number To Fractional String(number=w3948, width (-)=i16 6, precision (6)=i16 2) -> (F-format string=w3937:string)  [unwired: 1 in]
            n3000 = Number To Fractional String(number=w3947, width (-)=i16 6, precision (6)=i16 2) -> (F-format string=w3950:string)  [unwired: 1 in]
            n3001 = Number To Fractional String(number=w3963, width (-)=i16 6, precision (6)=i16 2) -> (F-format string=w3968:string)  [unwired: 1 in]
            n3002 = Number To Fractional String(number=w3952, width (-)=i16 6, precision (6)=i16 2) -> (F-format string=w3954:string)  [unwired: 1 in]
            n3003 = Number To Fractional String(number=w3938, width (-)=i16 6, precision (6)=i16 2) -> (F-format string=w3939:string)  [unwired: 1 in]
            n3004 = Number To Fractional String(number=w3951, width (-)=i16 6, precision (6)=i16 2) -> (F-format string=w3953:string)  [unwired: 1 in]
            n3005 = Number To Fractional String(number=w3934, width (-)=i16 6, precision (6)=i16 2) -> (F-format string=w3933:string)  [unwired: 1 in]
            n3006 = Number To Fractional String(number=w3930, precision (6)=i16 2) -> (F-format string=w3929:string)  [unwired: 2 in]
            n3007 = call-dynamic "Set Report Header Text.vi"("report in"=w3972, "center header text"=w3924, "error in (no error)"=w3971) -> ("report out"=w3943:refnum<class "NI_report.lvclass">, "error out"=w3944:errorcluster)  [unwired: 11 in]
            n3008 = Concatenate Strings(w3932, w3916, w3968, w3932, w3913, w3937, w3932, w3911, w3950, w3932, w3908, w3939, w3932, w3904, w3954, w3932, w3901, w3953, w3932, w3899, w3933, w3932, w3896, w3929) -> (w3920:string)
            "export 2" <- w3920
            n3009 = call-poly <vilib>:"Append Report Text.vi"("report in"=w3943, "text"=w3942, "error in (no error)"=w3944) -> ("report out"=w3946:refnum<class "NI_report.lvclass">, "error out"=w3945:errorcluster)  [unwired: 9 in, 2 out]
            n3010 = local read "test by"() -> (w3919:string)
            n3011 = local read "TITTLE"() -> (w3921:string)
            n3012 = call-poly <vilib>:"Append Report Text.vi"("report in"=w3946, "error in (no error)"=w3945) -> ("report out"=w3967:refnum<class "NI_report.lvclass">, "error out"=w3965:errorcluster)  [unwired: 10 in, 2 out]
            n3013 = Concatenate Strings(w3921, w3920, w3919) -> (→"output":string)
            n3014 = call-poly <vilib>:"Append Report Text.vi"("report in"=w3967, "text"=w3920, "error in (no error)"=w3965) -> ("report out"=w3966:refnum<class "NI_report.lvclass">, "error out"=w3964:errorcluster)  [unwired: 9 in, 2 out]
            n3015 = call-dynamic "Print Report.vi"("report in"=w3966, "printer name (default)"=w3974, "error in (no error)"=w3964) -> ("report out"=w3976:refnum<class "NI_report.lvclass">, "error out"=w3977:errorcluster)  [unwired: 11 in]
            n3016 = call-dynamic "Dispose Report.vi"("report in"=w3976, "error in (no error)"=w3977) -> ()  [unwired: 13 in, 1 out]
          }
        }
        n3017 = case shown="True" "Print 2" {
          frame False {
          }
          frame True {
            n3018 = flat-sequence {
              frame #0 {
                n3019 = local read "s.NO"() -> (→"s.NO 2":string)
                n3020 = Wait (ms)(milliseconds to wait=u32 20) -> ()  [unwired: 1 out]
                n3021 = local read "Sample ID  3"() -> (→"Sample ID  6":string)
                n3022 = local read "Sample ID  4"() -> (→"Sample ID  7":string)
                n3023 = local read "Sample ID"() -> (→"Sample ID  2":string)
                n3024 = local read "Tested by"() -> (→"Tested by 2":string)
                n3025 = local read "Test Date"() -> (→"Test Date 2":string)
                n3026 = local read "Humidity after test 3"() -> (→"Humidity after test 4":dbl)
                n3027 = local read "Ref A Test Date :"() -> (→"TITTLE 4":string)
                n3028 = local read "Temperature before test 3"() -> (w3799:dbl)
                n3029 = local read "Temperature before test 3"() -> (→"Temperature after test 5":dbl)
                n3030 = local read "Temperature after test 3"() -> (→"Temperature after test 4":dbl)
                n3031 = local read "Humidity before test 3"() -> (→"Humidity before test 4":dbl)
                n3032 = local write "Temperature before test 3"(w3799) -> ()
                n3033 = local read "image data"() -> (w3790:T16)
                n3034 = String To Path(string="C:\\LAB-IQ\\im\\Temp_resized.jpg") -> (path=w3791:path)
                "path 2" <- w3791
                n3035 = call <vilib>:"Write JPEG File.vi"("image data"=w3790, "path to JPEG file"=w3791) -> ()  [unwired: 8 in, 2 out]
                "Ref A Test Date :" <- "Ref A Test Date :"
                "Ref B Test Date :" <- "Ref B Test Date :"
                "Ref B Scar Value :" <- "Ref B Scar Value :"
                "Ref A Scar Value :" <- "Ref A Scar Value :"
              }
              frame #1 {
                (unwired) HTML_Report_Image_Alignment."MIDDLE" ("alignment (default)")
                w3827 = u16 0 items=["portrait", "landscape"] ("orientation (portrait)")
                (unwired) HTML_Report_Image_Alignment."ABSMIDDLE" ("alignment (default)")
                (unwired) "TESTED BY : "
                (unwired) "TESTED DATE :"
                (unwired) "SAMPLE ID : "
                (unwired) "SAMPLE DESIGN : "
                w3860 = "\r"
                # "add image"
                n3036 = Wait (ms)(milliseconds to wait=u32 20) -> ()  [unwired: 1 out]
                n3037 = local read "Sample ID  2"() -> (w3853:string)
                n3038 = local read "Wear Scar X"() -> (w3825:dbl)
                "Length ( microns ) 2" <- w3825
                n3039 = local read "Wear Scar Y"() -> (w3824:dbl)
                "Wear Scar Y ( microns ) :" <- w3824
                n3040 = local read "Test Date 2"() -> (w3854:string)
                n3041 = local read "Tested by 2"() -> (w3855:string)
                n3042 = local read "String 46"() -> (w3851:string)
                n3043 = local read "String 48"() -> (w3857:string)
                n3044 = local read "String 47"() -> (w3856:string)
                n3045 = local read "String 49"() -> (w3858:string)
                n3046 = local read "String 10"() -> (w3811:string)
                n3047 = local read "s.NO 2"() -> (w3852:string)
                n3048 = Add(x=w3825, y=w3824) -> (x+y=w3823:dbl)
                n3049 = call <vilib>:"New Report.vi"("report type"=enum16{"Standard Report", "HTML"}."HTML") -> ("report out"=w3831:refnum<class "NI_report.lvclass">, "error out"=w3829:errorcluster)  [unwired: 13 in]
                n3050 = Concatenate Strings(w3860, w3851, w3852, w3860, w3857, w3853, w3860, w3856, w3854, w3860, w3858, w3855, w3860) -> (→"test by 2":string)
                n3051 = Concatenate Strings("C:\\LAB-IQ\\Data\\" ("string"), w3811, ".jpg" ("string")) -> ()  [unwired: 1 out]
                n3052 = Divide(x=w3823, y=2.0) -> (x/y=→"Mean Wear ( microns) :":dbl)
                n3053 = call-dynamic "Set Report Orientation.vi"("report in"=w3831, "orientation (portrait)"=w3827, "error in (no error)"=w3829) -> ("report out"=w3830:refnum<class "NI_report.lvclass">, "error out"=w3828:errorcluster)  [unwired: 11 in]
                n3054 = for {
                  N: 5 -> [_]
                  tunnel: w3830 -> [w3881]
                  tunnel: [w3880] -> w3809
                  tunnel: w3828 -> [w3879]
                  tunnel: [w3878] -> w3808
                  n3055 = call-dynamic "Set Report Tab Width.vi"("report in"=w3881, "error in (no error)"=w3879) -> ("report out"=w3880:refnum<class "NI_report.lvclass">, "error out"=w3878:errorcluster)  [unwired: 12 in]
                }
                n3056 = local read "TITTLE"() -> (w3826:string)
                n3057 = call-dynamic "Set Report Header Text.vi"("report in"=w3809, "center header text"=w3826, "error in (no error)"=w3808) -> ("report out"=w3847:refnum<class "NI_report.lvclass">, "error out"=w3846:errorcluster)  [unwired: 11 in]
                n3058 = for {
                  N: 1 -> [_]
                  tunnel: [w3885] -> w3833
                  tunnel: [w3884] -> w3832
                  tunnel: w3847 -> [w3883]
                  tunnel: w3846 -> [w3882]
                  n3059 = call-dynamic "New Report Line.vi"("report in"=w3883, "error in (no error)"=w3882) -> ("report out"=w3885:refnum<class "NI_report.lvclass">, "error out"=w3884:errorcluster)  [unwired: 12 in]
                }
                n3060 = for {
                  N: 2 -> [_]
                  tunnel: [w3877] -> w3839
                  tunnel: [w3876] -> w3838
                  tunnel: w3833 -> [w3875]
                  tunnel: w3832 -> [w3874]
                  n3061 = call-dynamic "New Report Line.vi"("report in"=w3875, "error in (no error)"=w3874) -> ("report out"=w3877:refnum<class "NI_report.lvclass">, "error out"=w3876:errorcluster)  [unwired: 12 in]
                }
                n3062 = for {
                  N: 25 -> [_]
                  tunnel: w3839 -> [w3873]
                  tunnel: w3838 -> [w3871]
                  tunnel: [w3872] -> w3842
                  tunnel: [w3870] -> w3841
                  n3063 = call-dynamic "Set Report Tab Width.vi"("report in"=w3873, "error in (no error)"=w3871) -> ("report out"=w3872:refnum<class "NI_report.lvclass">, "error out"=w3870:errorcluster)  [unwired: 12 in]